vi "Main.vi"() -> ()   [LabVIEW 2020]
uses:
  System.Windows.Forms
  Global_Variable/Global.vi
  Global_Variable/A180648.vi
  <userlib>/_MGI/Menu Building/MenuTypes/MenuStrip/MGI_MenuStrip.lvclass
  <userlib>/_MGI/Menu Building/MenuItemStatusChange/MGI_MenuItemStatusChange.lvclass
  Libraries/S7/S7.lvlib
panel:
  out "状态":string
  out "客户软件版本号":string
  in  "Andon":enum32{"未选择", "缺料报警", "质量报警", "故障报警"}(radio)
  out "PLC":bool
  in  "菜单":refnum<k24>(container)
  in  "Result":string[][](table)
  out "逆向空载":bool
  out "试验计时":u16
  out "产品编号":string
  out "生产数量":i32
  out "合格数量":i32
  out "userStatus":string caption="用户状态"
  out "userName":string caption="用户名"
  out "connectionMode":string caption="联机类型"
  out "产品型号":string
  out "侧铆":bool
  out "轴承压装":bool
  out "振动NVH":bool
  out "磨合":bool
  out "备用试验2":bool
  out "传感器特性":bool
  out "电流特性":bool
  out "端铆":bool
  in  "更换产品":refnum<vi>
  out "提示信息":string
  out "错误":bool
  out "时间字符串":string
  out "日期字符串":string
  out "自动":bool=TRUE
  # "上柱管组件装配"
  # "试验项目"
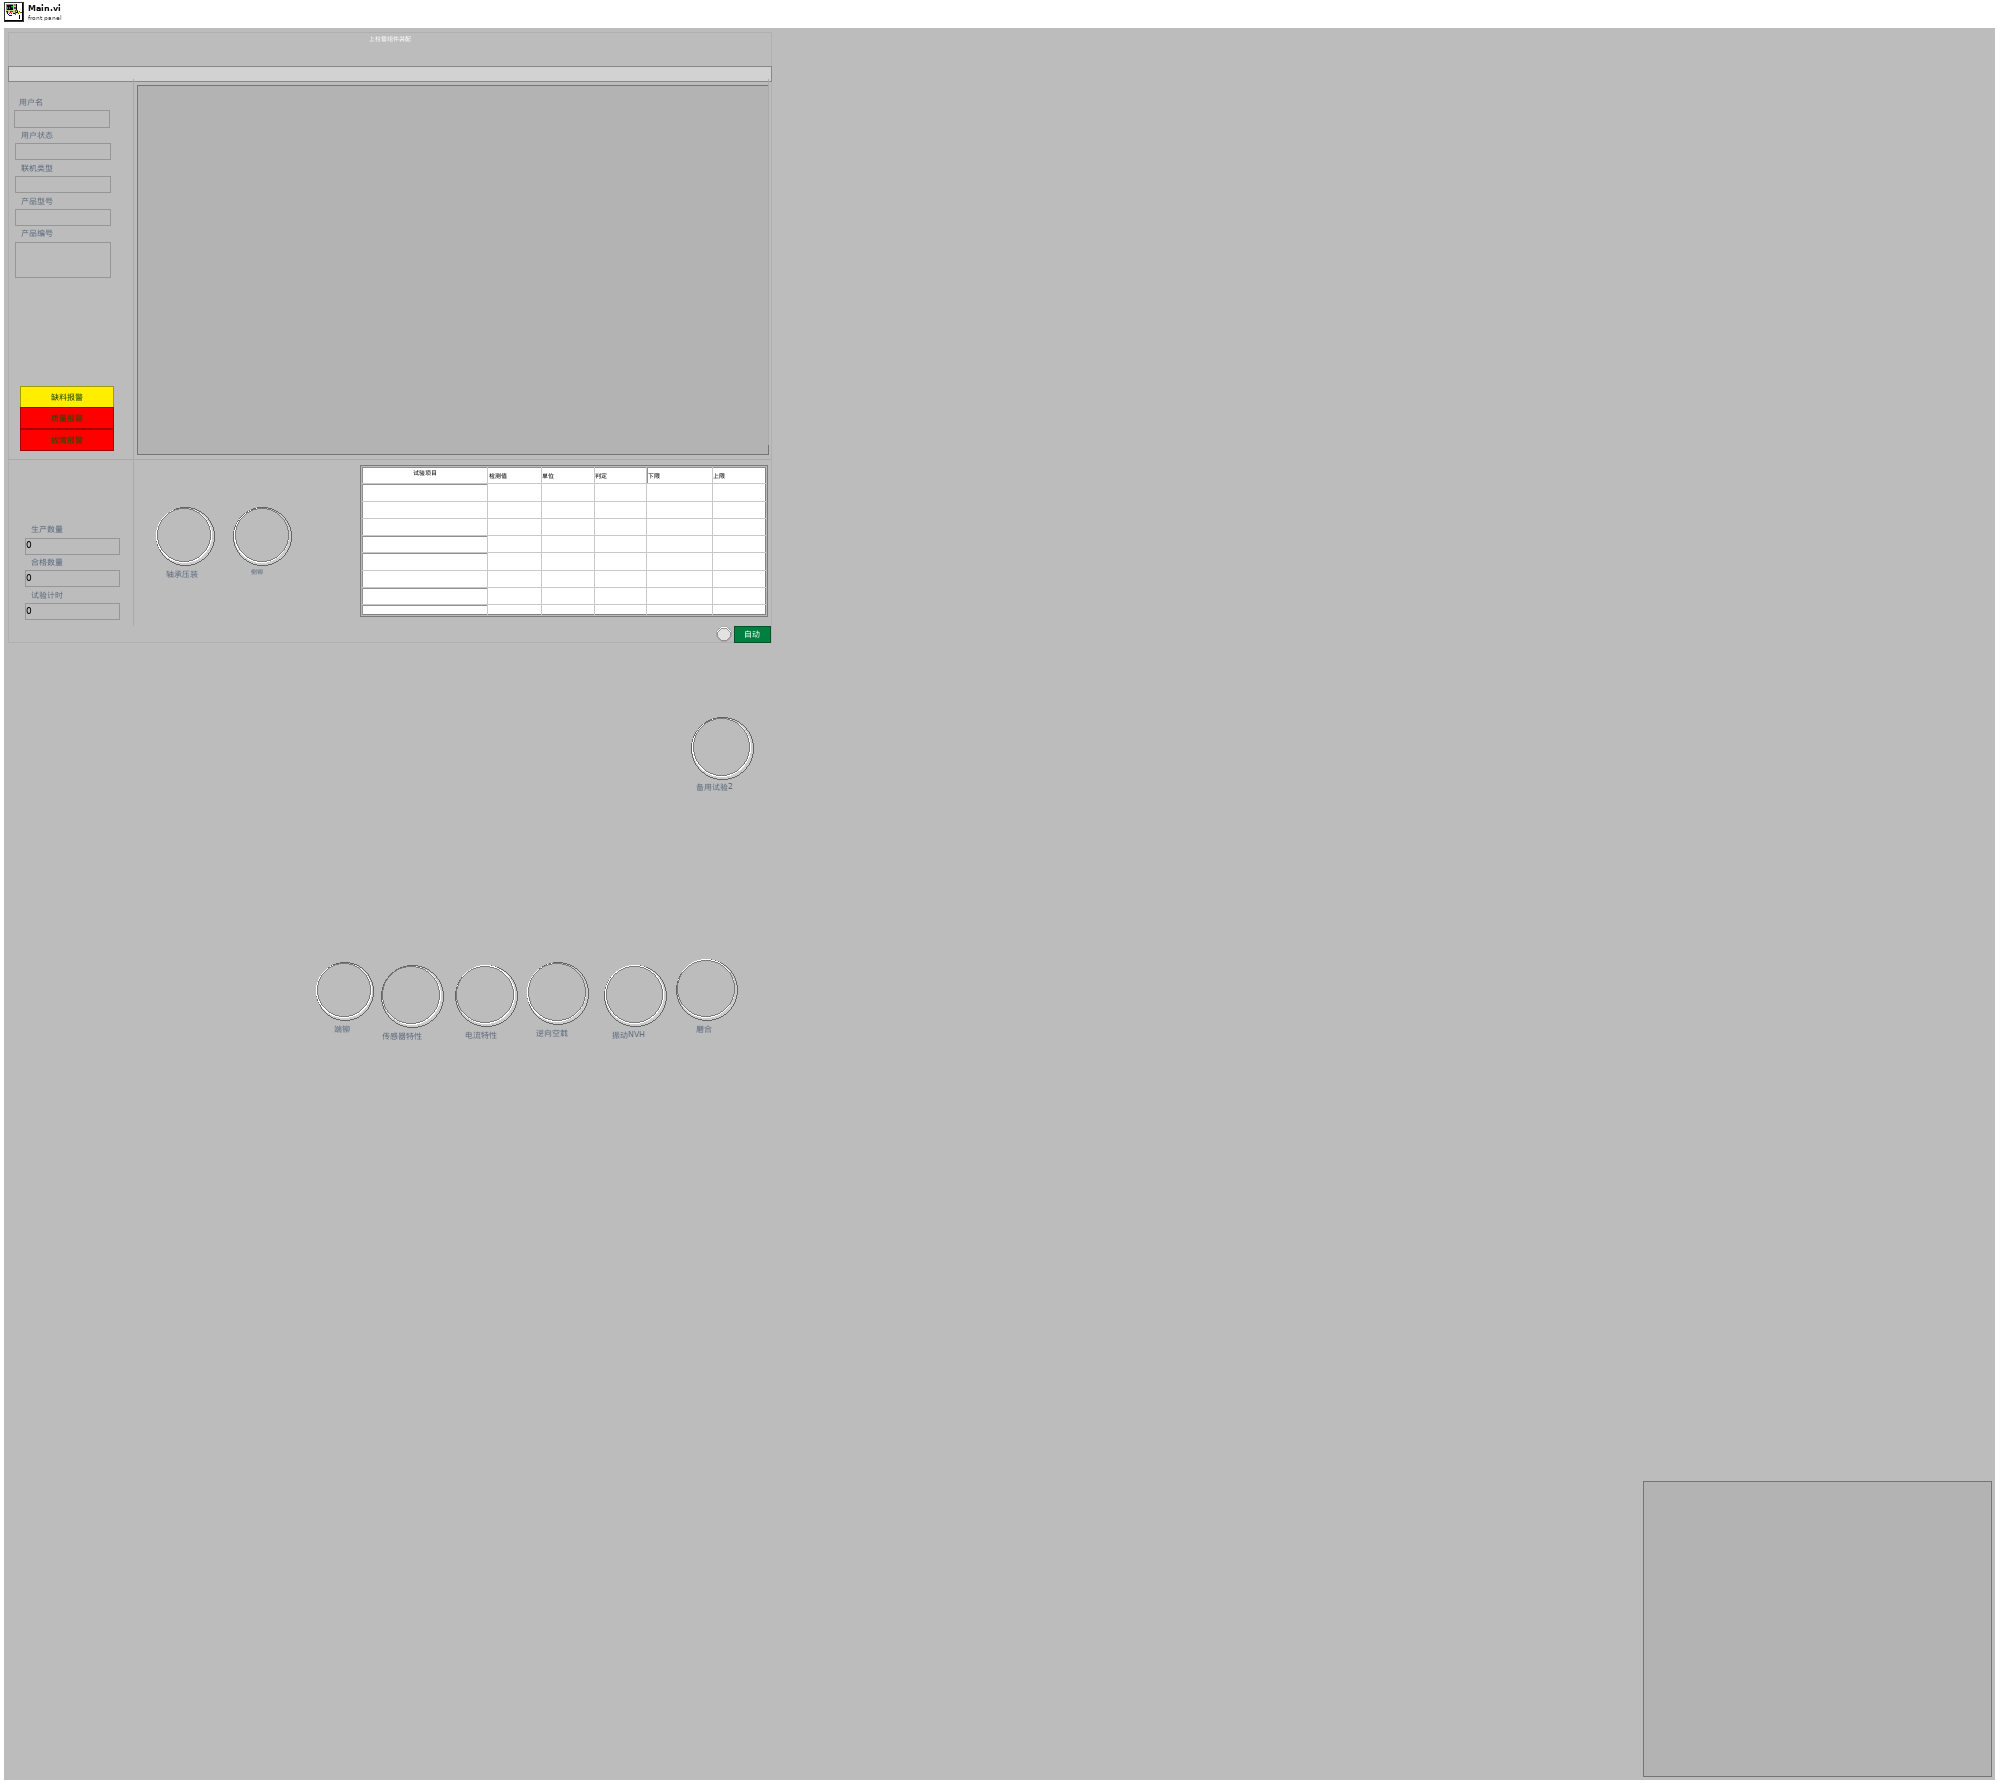
[diagram p1: front panel]
types:
  T1 = typedef "S7.lvlib/Broadcast Events--cluster.ctl" = cluster{"Module Did Init":refnum<user-event>, "Status Updated":refnum<user-event>, "Error Reported":refnum<user-event>, "Module Did Stop":refnum<user-event>, "Update Module Execution Status":refnum<user-event>}
  T2 = enum32{"轴承压装", "侧铆", "端铆", "力特性", "电流特性", "传感器特性", "逆向空载", "磨合"}
  T3 = enum32{"Invalid", "Standard", "Closed", "Hidden", "Minimized", "Maximized"}
  T4 = cluster{"设备名称":string, "操作人员":string, "设备状态":enum16{"设备离线", "设备正常", "设备缺料", "设备故障", "质量报警"}, "附加信息":string}
  T5 = enum32{"invalid app kind", "Development System", "Run Time System", "Student Edition", "Embedded LabVIEW", "Evaluation", "Custom"}
  T6 = cluster{"操作员编号":string, "操作员姓名":string, "操作员权限":string, "联机模式":enum16{"单机", "追溯"}}
  T7 = cluster{"Core":cluster{"Current VI Reference":refnum<vi>, "Close Panel on Exit?":bool}, "Your Boolean data":bool, "Your string data":string}
  T8 = cluster{"Current VI Reference":refnum<vi>, "Close Panel on Exit?":bool}
  T9 = cluster{"用户编号":string, "用户名":string, "用户密码(密文)":string, "用户权限":string}
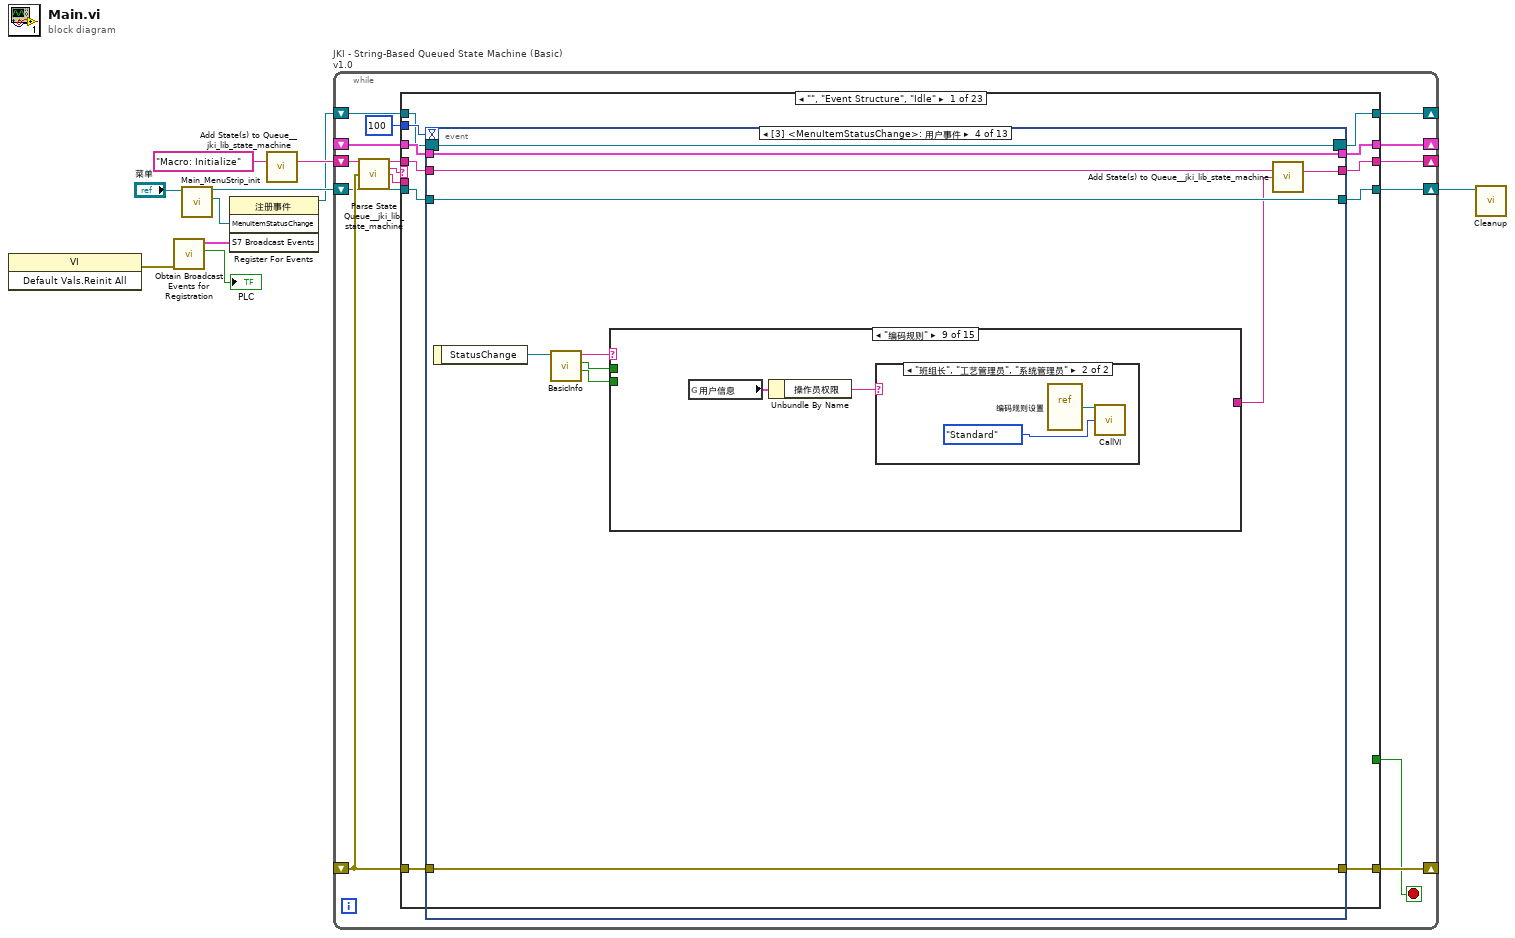
[diagram p0: block diagram]
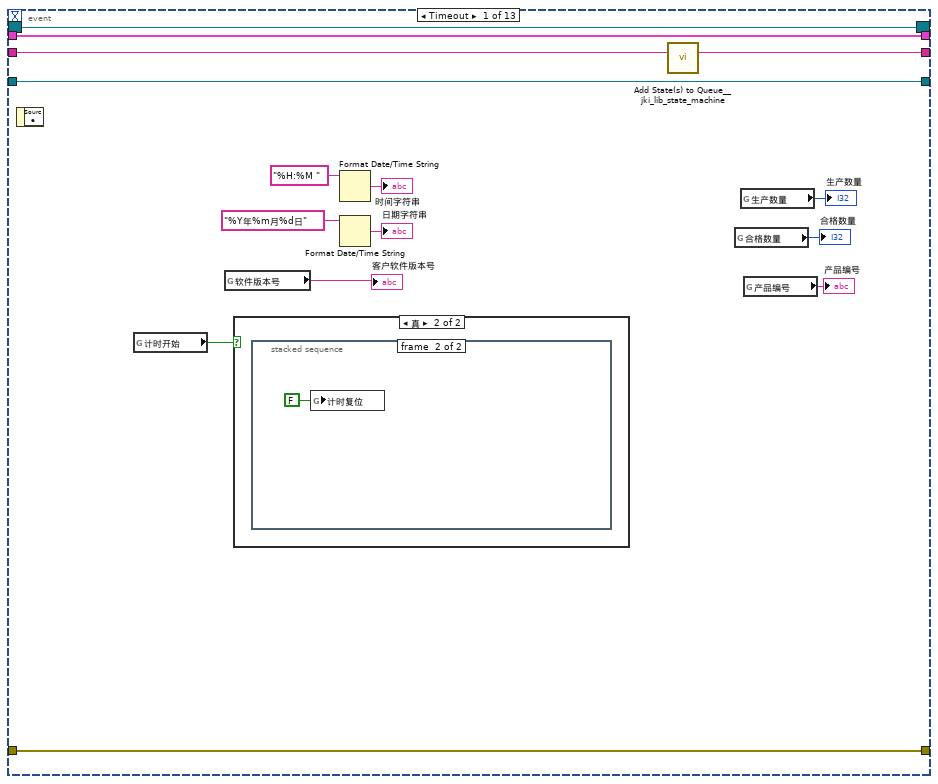
[diagram p2: hidden frame]
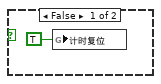
[diagram p3: hidden frame]
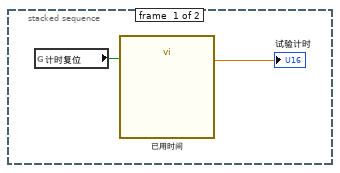
[diagram p4: hidden frame]
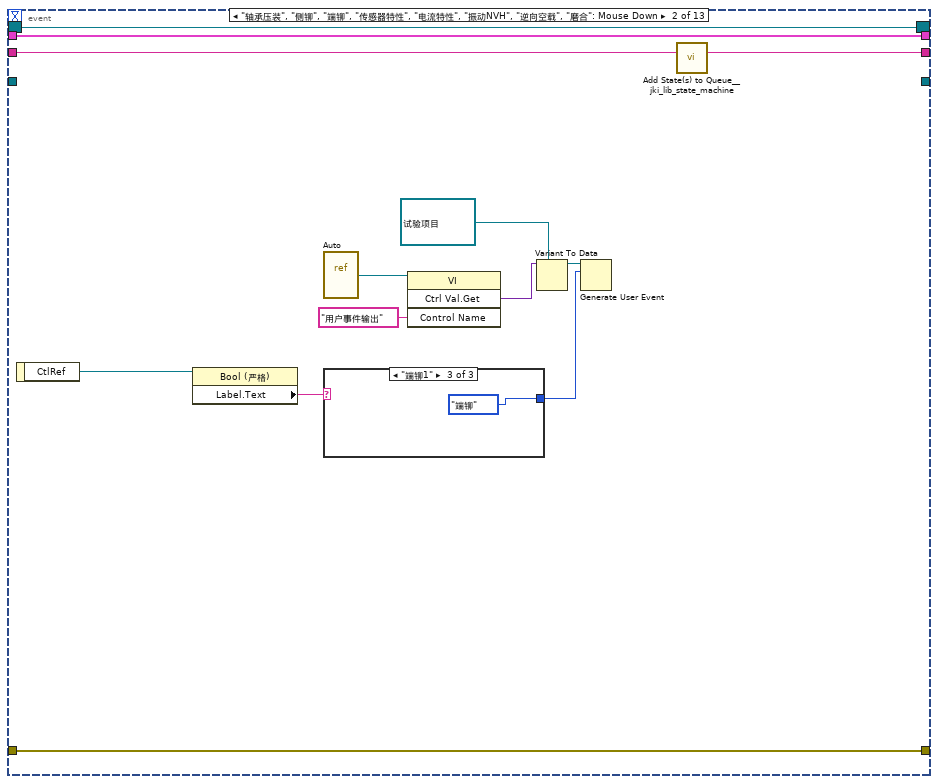
[diagram p5: hidden frame]
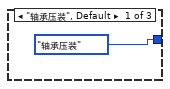
[diagram p6: hidden frame]
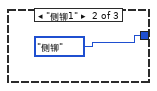
[diagram p7: hidden frame]
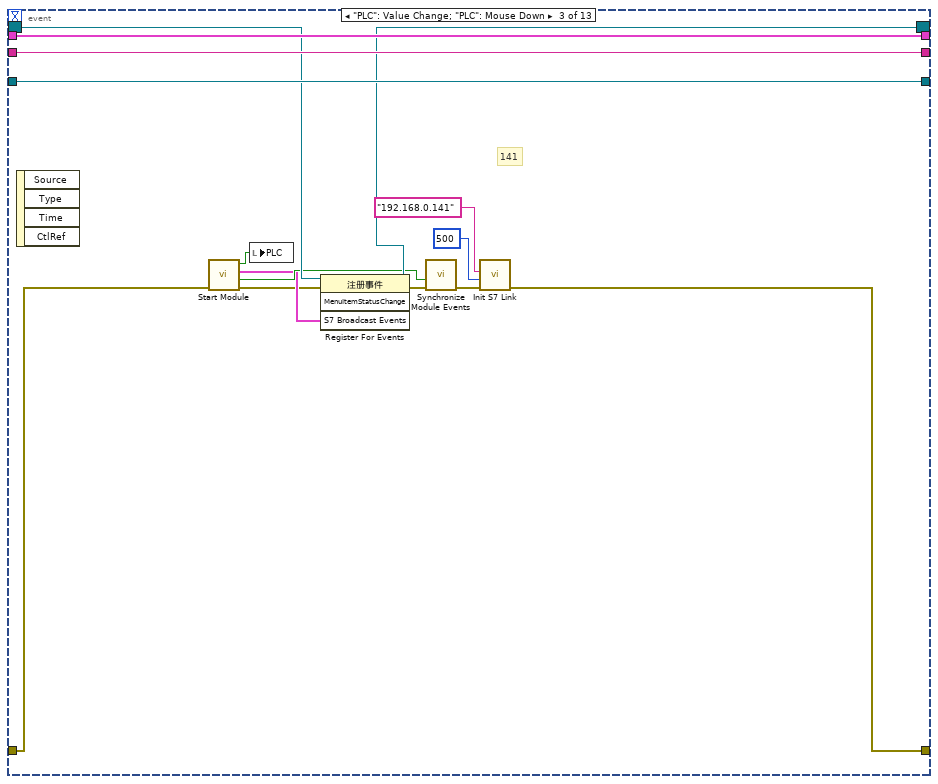
[diagram p8: hidden frame]
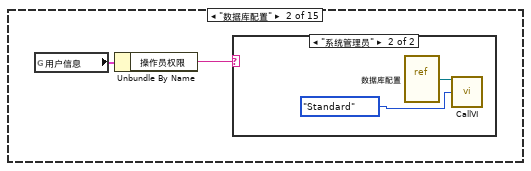
[diagram p10: hidden frame]
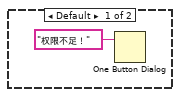
[diagram p11: hidden frame]
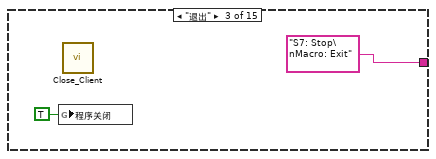
[diagram p12: hidden frame]
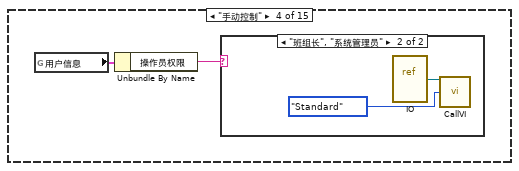
[diagram p13: hidden frame]
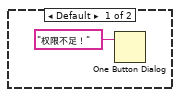
[diagram p14: hidden frame]
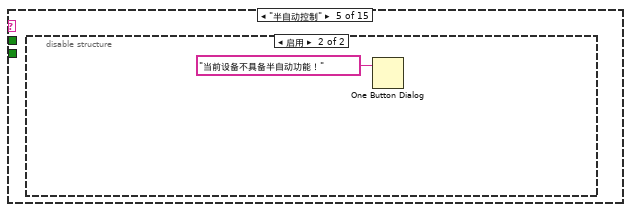
[diagram p15: hidden frame]
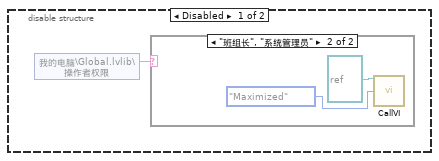
[diagram p16: hidden frame]
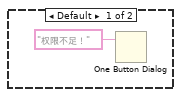
[diagram p17: hidden frame]
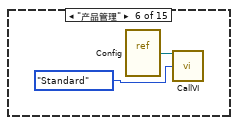
[diagram p18: hidden frame]
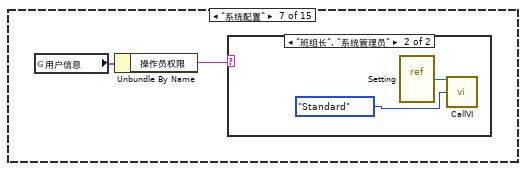
[diagram p19: hidden frame]
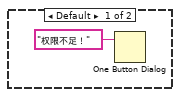
[diagram p20: hidden frame]
diagram:
  n1 = invoke class="VI" method="Default Vals.Reinit All"() -> (error out=w3:errorcluster)  [unwired: 3 in, 2 out]
  n2 = call "Obtain Broadcast Events for Registration.vi"("error in (no error)"=w3) -> ("Already running?"=→"PLC":bool, "S7 Broadcast Events"=w5:T1)  [unwired: 8 in, 1 out]
  n3 = call "Main_MenuStrip_init.vi"("MenuStrip"="菜单") -> ("MenuItemStatusChange"=w2:refnum<user-event>, "Menu out"=w7:refnum<class "MGI_MenuStrip.lvclass">)  [unwired: 9 in]
  n4 = register-events(w2, w5) -> (reference out=w1:refnum<event-registration>)  [unwired: 2 in, 1 out]
  n5 = call <vilib>:"Add State(s) to Queue__jki_lib_state_machine.vi"("State(s) in (\"\")"="Macro: Initialize") -> ("States Out"=w10:string)  [unwired: 14 in]
  n6 = while "JKI - String-Based Queued State Machine (Basic) v1.0" {
    shift-right: [w19] -> _
    shift-left: _ -> [w18]
    shift-right: [w21] -> _
    shift-left: _ -> [w16]
    shift-right: [w20] -> _
    shift-left: w10 -> [w22]
    shift-right: [w14] -> w6
    shift-left: w7 -> [w15]
    shift-right: [w12] -> _
    shift-left: w1 -> [w11]
    stop <- w13 stop-if-true
    n7 = call <vilib>:"Parse State Queue__jki_lib_state_machine.vi"("State Queue"=w22, "Error In (no error)"=w16) -> ("Remaining States"=w24:string, "Current State"=w25:string, "Arguments"=w23:string)  [unwired: 11 in]
    n8 = case shown="\"\", \"Event Structure\", \"Idle\"" w25 {
      selector: w25 -> [_ _ w273 _ _ _ _ _ _ _ _ _ _ _ _ _ _ _ _ _ _ _ _]
      tunnel: w24 -> [w36 w270 w277 w297 w305 w312 w318 w322 w328 w334 w340 w349 w360 w368 w374 w381 w395 w431 w439 w452 w480 w487 w499]
      tunnel: w23 -> [_ _ _ _ _ _ _ _ _ _ _ _ _ _ _ _ _ _ w434 w446 _ _ _]
      tunnel: w18 -> [w34 w267 w275 w288 w302 w310 w315 w323 w331 w337 w343 w346 _ w363 w371 w379 w393 w428 w437 w448 w477 w484 w496]
      tunnel: [w33 w268 w279 w294 errorcluster {"status"=FALSE, "code"=0, "source"=""} ("error out") w309 w316 w320 w326 w333 w339 w347 w357 w364 w372 w378 w391 w429 w435 w449 w478 w485 w497] -> w21
      tunnel: w16 -> [w32 w268 w278 w294 w301 w309 w316 w320 w327 w333 w339 w347 w357 w365 w372 w375 w391 w429 w436 w450 w478 w485 w497]
      tunnel: [w35 w269 w276 w296 w304 w311 w317 w322 w329 w335 w341 w348 w359 w367 w373 w380 w394 w430 w438 w451 w479 w486 w498] -> w20
      tunnel: [w31 w267 w275 w295 w302 w310 w315 w323 w331 w337 w343 w346 w358 w363 w371 w379 w393 w428 w437 w448 w477 w484 w496] -> w19
      tunnel: 100 ("Timeout") -> [w30 _ _ _ _ _ _ _ _ _ _ _ _ _ _ _ _ _ _ _ _ _ _]
      tunnel: w15 -> [w29 w266 w272 w285 w299 w308 w314 w321 w330 w336 w342 w345 w351 w362 w370 w377 w392 w427 w433 w445 w476 w482 w489]
      tunnel: [w28 w266 w272 w285 w299 w308 w314 w321 w330 w336 w342 w345 w351 w362 w370 w377 w392 w427 w433 w445 w476 w482 w489] -> w14
      tunnel: [_ _ _ _ _ TRUE _ _ _ _ _ _ _ _ _ _ _ _ _ _ _ _ _] -> w13
      tunnel: [w26 w265 w271 w284 w298 w306 w313 w324 w325 w332 w338 w344 w352 w361 w369 w376 w390 w424 w432 w444 w475 w481 w488] -> w12
      tunnel: w11 -> [w27 w265 w271 w284 w298 w306 w313 w324 w325 w332 w338 w344 w352 w361 w369 w376 w390 w424 w432 w444 w475 w481 w488]
      frame "", "Event Structure", "Idle" {
        n9 = event shown="[3] <MenuItemStatusChange>: 用户事件" {
          selector: w27 -> [w39 w64 w81 w87 w153 w160 w167 w174 w188 w200 w207 w215 _]
          dyn-events: [w39 w64 w80 w87 w153 w160 w167 w174 w188 w200 w207 w215 _] -> w26
          timeout: w30 -> [_ _ _ _ _ _ _ _ _ _ _ _ _]
          tunnel: w36 -> [w51 w67 w85 w96 w154 w161 w170 w177 w185 w204 w214 w217 w259]
          tunnel: [w50 w66 w85 w94 w155 w162 w171 w178 w186 w205 w213 w218 w259] -> w35
          tunnel: w34 -> [w49 w68 w86 w95 w157 w165 w172 w179 w187 w206 w211 w220 w260]
          tunnel: [w40 w65 w82 w97 w158 w163 w168 w180 w183 w203 w212 w219 w257] -> w33
          tunnel: w32 -> [w40 w65 w83 w97 w158 w163 w168 w181 w183 w203 w212 w219 w257]
          tunnel: [w49 w68 w86 w95 w157 w165 w172 w179 w187 w206 w211 w220 w260] -> w31
          tunnel: w29 -> [w38 _ w84 w90 w156 w164 w169 w176 w184 _ _ _ w258]
          tunnel: [w38 _ w84 w90 w156 w164 w169 w176 w184 _ _ _ w258] -> w28
          event Timeout {
            n10 = event-data() -> ()  [unwired: 1 in, 1 out]
            n11 = global read "Global.vi" "计时开始"() -> (w42:bool)
            n12 = global read "Global.vi" "软件版本号"() -> (→"客户软件版本号":string)
            n13 = case shown="真" w42 {
              frame False {
                n14 = global write "Global.vi" "计时复位"(TRUE ("计时复位")) -> ()
              }
              frame True {
                n15 = stacked-sequence {
                  frame #0 {
                    n16 = global read "Global.vi" "计时复位"() -> (w53:bool)
                    n17 = call "已用时间"("Reset"=w53) -> ("Elapsed Time (s)"=→"试验计时":dbl)  [unwired: 11 in, 7 out]
                  }
                  frame #1 {
                    n18 = global write "Global.vi" "计时复位"(FALSE ("计时复位")) -> ()
                  }
                }
              }
            }
            n19 = Format Date/Time String(time format string (%c)="%H:%M ") -> (date/time string=→"时间字符串":string)  [unwired: 2 in]
            n20 = Format Date/Time String(time format string (%c)="%Y年%m月%d日") -> (date/time string=→"日期字符串":string)  [unwired: 2 in]
            n21 = call <vilib>:"Add State(s) to Queue__jki_lib_state_machine.vi"("State(s) in (\"\")"=w51) -> ("States Out"=w50:string)  [unwired: 14 in]
            n22 = global read "Global.vi" "合格数量"() -> (→"合格数量":i32)
            n23 = global read "Global.vi" "生产数量"() -> (→"生产数量":i32)
            n24 = global read "Global.vi" "产品编号"() -> (→"产品编号":string)
          }
          event "轴承压装", "侧铆", "端铆", "传感器特性", "电流特性", "振动NVH", "逆向空载", "磨合": Mouse Down {
            w57 = refnum<user-event> refnum items=["轴承压装", "侧铆", "端铆", "力特性", "电流特性", "传感器特性", "逆向空载", "磨合"] ("用户事件输出")
            n25 = event-data() -> ("CtlRef"=w61:refnum<vi>)  [unwired: 1 in]
            n26 = property class="Bool (严格)"(reference=w61) -> ("Label.Text"=w60:string)  [unwired: 1 in, 2 out]
            n27 = vi-ref "Auto.vi"() -> (w63:refnum<vi>)
            n28 = case shown="\"端铆1\"" w60 {
              tunnel: [T2."轴承压装" ("试验项目") T2."侧铆" ("试验项目") T2."端铆" ("试验项目")] -> w59
              frame "轴承压装", Default {
              }
              frame "侧铆1" {
              }
              frame "端铆1" {
              }
            }
            n29 = invoke class="VI" method="Ctrl Val.Get"(reference=w63, "Control Name"="用户事件输出" ("控件名")) -> ("Get Control Value Variant"=w62:variant)  [unwired: 2 in, 3 out]
            n30 = Variant To Data(type=w57, Variant=w62) -> (data=w56:refnum<user-event>)  [unwired: 1 in, 1 out]
            n31 = Generate User Event(user event=w56, event data cluster=w59) -> ()  [unwired: 2 in, 2 out]
            n32 = call <vilib>:"Add State(s) to Queue__jki_lib_state_machine.vi"("State(s) in (\"\")"=w67) -> ("States Out"=w66:string)  [unwired: 14 in]
          }
          event "PLC": Value Change; "PLC": Mouse Down {
            # "141"
            n33 = event-data() -> ()  [unwired: 1 in, 4 out]
            n34 = call "Start Module.vi"("error in (no error)"=w83) -> ("error out"=w74:errorcluster, "Wait for Event Sync?"=w79:bool, "S7 Broadcast Events"=w78:T1, "Module Was Already Running?"=w77:bool)  [unwired: 7 in]
            n35 = local write "PLC"(w77) -> ()
            n36 = register-events(reference=w81, error in=w74, w78) -> (reference out=w80:refnum<event-registration>, error out=w73:errorcluster)  [unwired: 1 in]
            n37 = call "Synchronize Module Events.vi"("error in (no error)"=w73, "Wait for Event Sync?"=w79) -> ("error out"=w72:errorcluster)  [unwired: 9 in]
            n38 = call "Init S7 Link.vi"("error in (no error)"=w72, "超时"=500, "IP"="192.168.0.141") -> ("error out"=w82:errorcluster)  [unwired: 8 in]
          }
          event User Event {
            n39 = event-data() -> ("StatusChange"=w88:refnum<class "MGI_MenuItemStatusChange.lvclass">)  [unwired: 1 in]
            n40 = call <userlib>:"BasicInfo.vi"("MGI_MenuItemStatusChange in"=w88) -> ("Enabled?"=w91:bool, "Checked?"=w92:bool, "Tag"=w93:string)  [unwired: 7 in, 1 out]
            n41 = case shown="\"编码规则\"" w93 {
              tunnel: w92 -> [_ _ _ _ _ _ _ _ _ _ _ _ _ _ _]
              tunnel: w91 -> [_ _ _ _ _ _ _ _ _ _ _ _ _ _ _]
              tunnel: [_ _ "S7: Stop\nMacro: Exit" _ _ _ _ _ _ _ _ _ _ _ _] -> w89
              frame "假", Default {
              }
              frame "数据库配置" {
                n42 = global read "用户信息.vi" "用户信息"() -> (w99:T6)
                n43 = Unbundle By Name(w99) -> ("操作员权限"=w98:string)
                n44 = case shown="\"系统管理员\"" w98 {
                  frame Default {
                    n45 = One Button Dialog(message="权限不足！" ("消息")) -> ()  [unwired: 1 in, 1 out]
                  }
                  frame "系统管理员" {
                    n46 = vi-ref "数据库配置.vi"() -> (w102:refnum<vi>)
                    n47 = call "CallVI.vi"("VI引用"=w102, "状态"=T3."Standard") -> ()  [unwired: 12 in, 2 out]
                  }
                }
              }
              frame "退出" {
                n48 = global write "Global.vi" "程序关闭"(TRUE ("程序关闭")) -> ()
                n49 = call "Close_Client.vi"() -> ()  [unwired: 12 in]
              }
              frame "手动控制" {
                n50 = global read "用户信息.vi" "用户信息"() -> (w106:T6)
                n51 = Unbundle By Name(w106) -> ("操作员权限"=w105:string)
                n52 = case shown="\"班组长\", \"系统管理员\"" w105 {
                  frame Default {
                    n53 = One Button Dialog(message="权限不足！" ("消息")) -> ()  [unwired: 1 in, 1 out]
                  }
                  frame "班组长", "系统管理员" {
                    n54 = vi-ref "IO.vi"() -> (w109:refnum<vi>)
                    n55 = call "CallVI.vi"("VI引用"=w109, "状态"=T3."Standard") -> ()  [unwired: 12 in, 2 out]
                  }
                }
              }
              frame "半自动控制" {
                n56 = disable-structure shown="启用" {
                  frame Disabled {
                    n57 = shared-variable "我的电脑\\Global.lvlib\\操作者权限"() -> (w110:string)  [unwired: 1 in, 1 out]
                    n58 = case shown="\"班组长\", \"系统管理员\"" w110 {
                      frame Default {
                        n59 = One Button Dialog(message="权限不足！" ("消息")) -> ()  [unwired: 1 in, 1 out]
                      }
                      frame "班组长", "系统管理员" {
                        n60 = call "CallVI.vi"("VI引用"=refnum<vi> refnum, "状态"=T3."Maximized") -> ()  [unwired: 12 in, 2 out]
                      }
                    }
                  }
                  frame Enabled {
                    n61 = One Button Dialog(message="当前设备不具备半自动功能！" ("消息")) -> ()  [unwired: 1 in, 1 out]
                  }
                }
              }
              frame "产品管理" {
                n62 = vi-ref "Config.vi"() -> (w116:refnum<vi>)
                n63 = call "CallVI.vi"("VI引用"=w116, "状态"=T3."Standard") -> ()  [unwired: 12 in, 2 out]
              }
              frame "系统配置" {
                n64 = global read "用户信息.vi" "用户信息"() -> (w118:T6)
                n65 = Unbundle By Name(w118) -> ("操作员权限"=w117:string)
                n66 = case shown="\"班组长\", \"系统管理员\"" w117 {
                  frame Default {
                    n67 = One Button Dialog(message="权限不足！" ("消息")) -> ()  [unwired: 1 in, 1 out]
                  }
                  frame "班组长", "系统管理员" {
                    n68 = vi-ref "Setting.vi"() -> (w121:refnum<vi>)
                    n69 = call "CallVI.vi"("VI引用"=w121, "状态"=T3."Standard") -> ()  [unwired: 12 in, 2 out]
                  }
                }
              }
              frame "用户管理" {
                n70 = global read "用户信息.vi" "用户信息"() -> (w123:T6)
                n71 = Unbundle By Name(w123) -> ("操作员权限"=w122:string)
                n72 = case shown="\"系统管理员\"" w122 {
                  frame Default {
                    n73 = One Button Dialog(message="权限不足！" ("消息")) -> ()  [unwired: 1 in, 1 out]
                  }
                  frame "系统管理员" {
                    n74 = vi-ref "User_manager.vi"() -> (w126:refnum<vi>)
                    n75 = call "CallVI.vi"("VI引用"=w126, "状态"=T3."Standard") -> ()  [unwired: 12 in, 2 out]
                  }
                }
              }
              frame "编码规则" {
                n76 = global read "用户信息.vi" "用户信息"() -> (w128:T6)
                n77 = Unbundle By Name(w128) -> ("操作员权限"=w127:string)
                n78 = case shown="\"班组长\", \"工艺管理员\", \"系统管理员\"" w127 {
                  frame Default {
                    n79 = One Button Dialog(message="权限不足！" ("消息")) -> ()  [unwired: 1 in, 1 out]
                  }
                  frame "班组长", "工艺管理员", "系统管理员" {
                    n80 = vi-ref "编码规则设置.vi"() -> (w131:refnum<vi>)
                    n81 = call "CallVI.vi"("VI引用"=w131, "状态"=T3."Standard") -> ()  [unwired: 12 in, 2 out]
                  }
                }
              }
              frame "易损件管理" {
                n82 = vi-ref "易损件管理.vi"() -> (w133:refnum<vi>)
                n83 = call "CallVI.vi"("VI引用"=w133, "状态"=T3."Standard") -> ()  [unwired: 12 in, 2 out]
              }
              frame "物料批次管理" {
                n84 = vi-ref "批次管理.vi"() -> (w135:refnum<vi>)
                n85 = call "CallVI.vi"("VI引用"=w135, "状态"=T3."Standard") -> ()  [unwired: 12 in, 2 out]
              }
              frame "报表" {
                n86 = call "文件对话框"("start path"=path "D:/report", "prompt"="打开报表", "pattern (all files)"="*.doc;*.docx", "pattern label"="Word 文档") -> ("selected path"=w136:path, "error out"=w137:errorcluster)  [unwired: 8 in, 2 out]
                n87 = case shown="无错误" w137 {
                  selector: w137 -> [w143 w145]
                  tunnel: w136 -> [w144 _]
                  frame No Error {
                    w142 = 1 items=["Normal", "Maximize", "Minimize"] ("cpubbs_WindowState")
                    n88 = call "Open_Word.vi"("File Path"=w144, "cpubbs_WindowState"=w142, "错误输入（无错误）"=w143) -> ()  [unwired: 12 in, 1 out]
                  }
                  frame Error {
                    n89 = call <vilib>:"Clear Errors.vi"("error in (no error)"=w145) -> ()  [unwired: 5 in, 2 out]
                  }
                }
              }
              frame "报警信息" {
                n90 = vi-ref "报警信息.vi"() -> (w147:refnum<vi>)
                n91 = call "CallVI.vi"("VI引用"=w147, "状态"=T3."Standard") -> ()  [unwired: 12 in, 2 out]
              }
              frame "关于" {
                n92 = vi-ref "About.vi"() -> (w149:refnum<vi>)
                n93 = call "CallVI.vi"("VI引用"=w149, "状态"=T3."Standard") -> ()  [unwired: 12 in, 2 out]
              }
              frame "操作演示" {
                n94 = call <vilib>:"Application Directory.vi"() -> ("Application Directory"=w152:path)
                n95 = Build Path(base path=w152, name or relative path="操作演示" ("名称或相对路径")) -> (appended path=w151:path)
                n96 = call "自动播放ppt.vi"("路径"=w151) -> ()  [unwired: 10 in, 1 out]
              }
            }
            n97 = call <vilib>:"Add State(s) to Queue__jki_lib_state_machine.vi"("State(s) in (\"\")"=w96, "State(s) at Back (\"\")"=w89) -> ("States Out"=w94:string)  [unwired: 13 in]
          }
          event User Event {
            n98 = event-data() -> ("Init?"=w159:bool)  [unwired: 1 in, 1 out]
            n99 = local write "PLC"(w159) -> ()
            n100 = call <vilib>:"Add State(s) to Queue__jki_lib_state_machine.vi"("State(s) in (\"\")"=w154) -> ("States Out"=w155:string)  [unwired: 14 in]
          }
          event User Event {
            n101 = event-data() -> ("Running?"=w166:bool)  [unwired: 1 in]
            n102 = local write "PLC"(w166) -> ()
            n103 = call <vilib>:"Add State(s) to Queue__jki_lib_state_machine.vi"("State(s) in (\"\")"=w161) -> ("States Out"=w162:string)  [unwired: 14 in]
          }
          event User Event {
            n104 = event-data() -> ()  [unwired: 1 in, 7 out]
            n105 = local write "PLC"(FALSE ("PLC")) -> ()
            n106 = call <vilib>:"Add State(s) to Queue__jki_lib_state_machine.vi"("State(s) in (\"\")"=w170) -> ("States Out"=w171:string)  [unwired: 14 in]
          }
          event User Event {
            n107 = event-data() -> ("Error"=w182:errorcluster)  [unwired: 1 in]
            n108 = Merge Errors(w182, w181) -> (w180:errorcluster)
            n109 = call <vilib>:"Add State(s) to Queue__jki_lib_state_machine.vi"("State(s) in Front (\"\")"="S7: Initialize\nIdle", "State(s) in (\"\")"=w177) -> ("States Out"=w178:string)  [unwired: 13 in]
          }
          event "自动": Mouse Down {
            n110 = event-data() -> ()  [unwired: 1 in, 1 out]
            n111 = disable-structure shown="禁用" {
              frame Disabled {
                n112 = local read "自动"() -> (w189:bool)
                n113 = case shown="真" w189 {
                  frame False {
                    n114 = call "设备状态.vi"() -> ("Status_Read"=w190:i16)  [unwired: 11 in]
                    n115 = case shown="5" w190 {
                      frame 0, Default {
                        n116 = One Button Dialog(message="请复位！" ("消息")) -> ()  [unwired: 1 in, 1 out]
                      }
                      frame 5 {
                        n117 = vi-ref "Auto.vi"() -> (w194:refnum<vi>)
                        n118 = invoke class="VI" method="Ctrl Val.Set"(reference=w194, "Control Name"="STEP" ("控件名"), "Value"="进入自动" ("控件名")) -> ()  [unwired: 2 in, 5 out]
                      }
                    }
                  }
                  frame True {
                    n119 = Two Button Dialog(message="确定要退出自动？" ("消息")) -> (T button?=w195:bool)  [unwired: 2 in]
                    n120 = case shown="真" w195 {
                      frame False {
                      }
                      frame True {
                        n121 = vi-ref "Auto.vi"() -> (w199:refnum<vi>)
                        n122 = invoke class="VI" method="Ctrl Val.Set"(reference=w199, "Control Name"="STEP" ("控件名"), "Value"="退出自动" ("控件名")) -> ()  [unwired: 2 in, 5 out]
                      }
                    }
                  }
                }
              }
              frame Enabled {
              }
            }
            n123 = call <vilib>:"Add State(s) to Queue__jki_lib_state_machine.vi"("State(s) in (\"\")"=w185) -> ("States Out"=w186:string)  [unwired: 14 in]
          }
          event "错误": Mouse Down {
            n124 = event-data() -> ()  [unwired: 1 in, 8 out]
            n125 = vi-ref "报警信息.vi"() -> (w202:refnum<vi>)
            n126 = call "CallVI.vi"("VI引用"=w202, "状态"=T3."Standard") -> ()  [unwired: 12 in, 2 out]
            n127 = call <vilib>:"Add State(s) to Queue__jki_lib_state_machine.vi"("State(s) in (\"\")"=w204) -> ("States Out"=w205:string)  [unwired: 14 in]
          }
          event Panel Close? {
            n128 = event-data() -> ()  [unwired: 1 in, 1 out]
            n129 = global write "Global.vi" "程序关闭"(TRUE ("程序关闭")) -> ()
            n130 = call <vilib>:"Add State(s) to Queue__jki_lib_state_machine.vi"("State(s) in Front (\"\")"="S7: Stop\nMacro: Exit", "State(s) in (\"\")"=w214) -> ("States Out"=w213:string)  [unwired: 13 in]
            n131 = event-data("Discard?"=TRUE) -> ()  [unwired: 1 in, 1 out]
          }
          event "更换产品": Value Change {
            n132 = event-data() -> ("NewVal"=w216:refnum<vi>)  [unwired: 1 in, 5 out]
            n133 = stacked-sequence {
              tunnel: w216 -> [w221]
              frame #0 {
                n134 = stacked-sequence {
                  tunnel: w221 -> [w229 _]
                  frame #0 {
                    n135 = disable-structure shown="禁用" {
                      disable-tunnel: w229 -> [w231 _]
                      frame Disabled {
                        n136 = control-ref of="子面板"() -> (w230:refnum<vi>)
                        n137 = call "Call_SubPanal.vi"("VI引用句柄"=w231, "SubPnl引用句柄"=w230) -> ()  [unwired: 9 in, 1 out]
                      }
                      frame Enabled {
                      }
                    }
                    n138 = vi-ref "Auto.vi"() -> (w228:refnum<vi>)
                    n139 = invoke class="VI" method="Ctrl Val.Get"(reference=w228, "Control Name"="产品变更_Event" ("控件名")) -> ("Get Control Value Variant"=w226:variant)  [unwired: 2 in, 3 out]
                    n140 = global read "Global.vi" "产品型号"() -> (w223:string)
                    n141 = Variant To Data(type=refnum<user-event> refnum ("产品变更_Event"), Variant=w226) -> (data=w224:refnum<user-event>, error out=w222:errorcluster)  [unwired: 1 in]
                    n142 = Generate User Event(user event=w224, event data cluster=w223, error in=w222) -> ()  [unwired: 1 in, 2 out]
                    n143 = local write "产品型号"(w223) -> ()
                  }
                  frame #1 {
                    n144 = control-ref of="轴承压装"() -> (w232:refnum<vi>)
                    n145 = control-ref of="侧铆"() -> (w233:refnum<vi>)
                    n146 = control-ref of="端铆"() -> (w234:refnum<vi>)
                    n147 = global read "Global.vi" "试验项目"() -> (w237:bool[])
                    n148 = Build Array(w232, w233, w234) -> (w236:refnum<vi>[])
                    n149 = for {
                      tunnel: w236 -> [w241] mode=indexing
                      tunnel: w237 -> [w242] mode=indexing
                      shift-right: [w238] -> _
                      shift-left: 2000 -> [w239]
                      i -> [w240]
                      n150 = case shown="真" w242 {
                        tunnel: w241 -> [w243 w251]
                        tunnel: w240 -> [_ _]
                        tunnel: w239 -> [w245 w248]
                        tunnel: [w245 w246] -> w238
                        frame False {
                          n151 = property class="Bool (严格)"(reference=w243, "Top"=2000) -> ()  [unwired: 1 in, 2 out]
                        }
                        frame True {
                          n152 = Add(x=w248, y=120) -> (x+y=w246:i32)
                          n153 = Bundle(w246, 1235) -> (w249:cluster{i32, i32})  [unwired: 1 in]
                          n154 = property class="Bool (严格)"(reference=w251, "Position"=w249) -> ()  [unwired: 1 in, 2 out]
                        }
                      }
                    }
                  }
                }
              }
            }
            n155 = call <vilib>:"Add State(s) to Queue__jki_lib_state_machine.vi"("State(s) in (\"\")"=w217) -> ("States Out"=w218:string)  [unwired: 14 in]
          }
          event "Andon": Value Change {
            n156 = event-data() -> ("NewVal"=w256:enum32{"未选择", "缺料报警", "质量报警", "故障报警"})  [unwired: 1 in]
            n157 = case shown="\"未选择\", 默认" w256 {
              tunnel: [enum16{"设备离线", "设备正常", "设备缺料", "设备故障", "质量报警"}."设备正常" ("设备状态") enum16{"设备离线", "设备正常", "设备缺料", "设备故障", "质量报警"}."设备缺料" ("设备状态") enum16{"设备离线", "设备正常", "设备缺料", "设备故障", "质量报警"}."质量报警" ("设备状态") enum16{"设备离线", "设备正常", "设备缺料", "设备故障", "质量报警"}."设备故障" ("设备状态")] -> w254
              frame "未选择", Default {
              }
              frame "缺料报警" {
              }
              frame "质量报警" {
              }
              frame "故障报警" {
              }
            }
            n158 = local read "userName"() -> (w253:string)
            n159 = Bundle By Name(cluster=T4 {"设备名称"="最终性能试验台1", "操作人员"="", "设备状态"=enum."设备离线", "附加信息"=""} ("设备信息"), "操作人员"=w253, "设备状态"=w254) -> (w252:T4)
            n160 = call "Change_Client.vi"("设备信息"=w252) -> ()  [unwired: 10 in, 1 out]
          }
        }
      }
      frame "---------- Core ----------" {
        n161 = call <vilib>:"Add State(s) to Queue__jki_lib_state_machine.vi"("State(s) in (\"\")"=w270) -> ("States Out"=w269:string)  [unwired: 14 in]
      }
      frame Default {
        w282 = 42 items=["No error", "Argument error", "Memory is full", "Out of zone", "End of file", "File already open", "Generic file I/O error", "File not found", "File permission error", "Disk is full", "Duplicate path", "Too many files open", "System feature not enabled", "Resource file not found", "Cannot add resource", "Resource not found", "Image not found", "Image memory error", "Pen does not exist", "Config type invalid", "Config token not found", "Config parse error", "Config memory error", "Bad external code format", "Bad external code offset", "External code not present", "Null window", "Destroy window error", "Null menu", "Print aborted", "Bad print record", "Print driver error", "Windows error during printing", "Memory error during printing", "Print dialog error", "Generic print error", "Invalid device refnum", "Device not found", "Device parameter error", "Device unit error", "Cannot open device", "Device call aborted", "Generic error", "Cancelled by user", "Object ID too low", "Object ID too high", "Object not in heap", "Unknown heap", "Unknown object (invalid DefProc)", "Unknown object (DefProc not in table)", "Message out of range", "Invalid (null) method", "Unknown message", "Manager call not supported", "Bad address", "Network operation in progress", "Network operation timed out", "Connection is busy", "Network attribute not supported", "Network error", "Address in use", "System out of memory", "Connection aborted", "Connection refused", "Not connected", "Already connected", "Connection closed", "Initialization error (interapplication manager)", "Bad occurrence", "Wait on unbound occurrence handler", "Occurrence queue overflow", "Datalog type conflict", "Unused", "Unrecognized type (interapplication manager)", "Memory corrupt", "Failed to make temporary DLL", "Old CIN version", "Drag socket not found", "Failed to load drop-object", "Failed to register OLE object", "Failed to release OLE object", "Format specifier type mismatch", "Unknown format specifier", "Too few format specifiers", "Too many format specifiers", "Scan failed", "Newer CIN version", "Error converting to variant", "Runtime menu error", "Password tampered", "Variant attribute not found", "Incompatible variant data type", "Event data is not available", "Event Store is not present", "Occurrence is not found", "Event Queue is not created", "Event info is not available", "Refnum passed is NULL", "Error retrieving Class GUID", "Error retrieving CoClass GUID", "Error retrieving TypeLib GUID.", "Bad built application magic bytes.", "Specific driver is different from the specific driver associated with the Logical Name.", "There is no session opened to the class driver.", "Max Error", "MAX - Error with config objects", "MAX - Error loading configuration", "MAX - Group not supported"]
        # "Current State"
        n162 = Format Into String(format string="Software Exception: Unhandled State \"%s\"." ("message"), error in=w278, w273) -> (resulting string=w281:string, error out=w280:errorcluster)  [unwired: 1 in]
        n163 = call <vilib>:"Error Cluster From Error Code.vi"("show call chain? (False)"=TRUE, "error in (no error)"=w280, "error message (\"\")"=w281, "error code (0)"=w282) -> ("error out"=w279:errorcluster)  [unwired: 5 in]
        n164 = call <vilib>:"Add State(s) to Queue__jki_lib_state_machine.vi"("State(s) in (\"\")"=w277) -> ("States Out"=w276:string)  [unwired: 14 in]
      }
      frame "Initialize Core Data" {
        # "originally closed?"
        # "exe?"
        n165 = property class="VI"() -> ("Front Panel.Open"=w293:bool)  [unwired: 2 in, 2 out]
        n166 = property class="App"() -> ("App.Kind"=w292:T5)  [unwired: 2 in, 2 out]
        n167 = control-ref of="Current VI Reference"() -> (w286:refnum<vi>)
        n168 = Not(x=w293) -> (.not. x?=w290:bool)
        n169 = Equal?(x=w292, y=T5."Run Time System" ("Application:Kind")) -> (x = y?=w289:bool)
        n170 = Or(x=w290, y=w289) -> (x .or. y?=w287:bool)
        n171 = Bundle By Name(cluster=w288, "Core.Current VI Reference"=w286, "Core.Close Panel on Exit?"=w287) -> (w295:T7)
        n172 = call <vilib>:"Add State(s) to Queue__jki_lib_state_machine.vi"("State(s) in (\"\")"=w297) -> ("States Out"=w296:string)  [unwired: 14 in]
      }
      frame "Error Handler" {
        n173 = call <vilib>:"General Error Handler.vi"("error in (no error)"=w301) -> ()  [unwired: 10 in, 5 out]
        n174 = call <vilib>:"Add State(s) to Queue__jki_lib_state_machine.vi"("State(s) in Front (\"\")"="/* Post Error States", "State(s) in (\"\")"=w305) -> ("States Out"=w304:string)  [unwired: 13 in]
      }
      frame "Exit" {
        n175 = call <vilib>:"Add State(s) to Queue__jki_lib_state_machine.vi"("State(s) in (\"\")"=w312) -> ("States Out"=w311:string)  [unwired: 14 in]
        n176 = Quit LabVIEW() -> ()  [unwired: 1 in]
      }
      frame "--------- Library --------" {
        n177 = call <vilib>:"Add State(s) to Queue__jki_lib_state_machine.vi"("State(s) in (\"\")"=w318) -> ("States Out"=w317:string)  [unwired: 14 in]
      }
      frame "S7: Initialize" {
        n178 = property on="PLC" class="Bool (严格)"("Val(Sgnl)"=FALSE ("值(信号)")) -> ()  [unwired: 2 in, 2 out]
      }
      frame "S7: Stop" {
        n179 = call "Stop Module.vi"("error in (no error)"=w327) -> ("error out"=w326:errorcluster)  [unwired: 10 in]
        n180 = call <vilib>:"Add State(s) to Queue__jki_lib_state_machine.vi"("State(s) in (\"\")"=w328) -> ("States Out"=w329:string)  [unwired: 14 in]
      }
      frame "CAN: Start" {
        n181 = call <vilib>:"Add State(s) to Queue__jki_lib_state_machine.vi"("State(s) in (\"\")"=w334) -> ("States Out"=w335:string)  [unwired: 14 in]
      }
      frame "CAN: Stop" {
        n182 = call <vilib>:"Add State(s) to Queue__jki_lib_state_machine.vi"("State(s) in (\"\")"=w340) -> ("States Out"=w341:string)  [unwired: 14 in]
      }
      frame "---------- Data ----------" {
        n183 = call <vilib>:"Add State(s) to Queue__jki_lib_state_machine.vi"("State(s) in (\"\")"=w349) -> ("States Out"=w348:string)  [unwired: 14 in]
      }
      frame "Data: Initialize" {
        w354 = T8 {"Current VI Reference"=refnum, "Close Panel on Exit?"=FALSE}  # Core
        w356 = TRUE  # Your Boolean data
        w355 = ""  # Your string data
        n184 = global write "Global.vi" "程序关闭"(FALSE ("程序关闭")) -> ()
        n185 = global write "Global.vi" "计时开始"(FALSE ("计时结束")) -> ()
        n186 = Bundle("Core"=w354, "Your Boolean data"=w356, "Your string data"=w355) -> (w358:T7)  [unwired: 1 in]
        n187 = call <vilib>:"Add State(s) to Queue__jki_lib_state_machine.vi"("State(s) in (\"\")"=w360) -> ("States Out"=w359:string)  [unwired: 14 in]
      }
      frame "Data: Cleanup" {
        n188 = Unbundle By Name(w363) -> ("Core.Current VI Reference"=w366:refnum<vi>)
        n189 = Close Reference(reference=w366, error in (no error)=w365) -> (error out=w364:errorcluster)
        n190 = call <vilib>:"Add State(s) to Queue__jki_lib_state_machine.vi"("State(s) in (\"\")"=w368) -> ("States Out"=w367:string)  [unwired: 14 in]
      }
      frame "---------- UI ----------" {
        # "Do not put any code in this frame.\n(It is a separator no-op. You can make a copy of this frame to create a new UI frame)"
        n191 = call <vilib>:"Add State(s) to Queue__jki_lib_state_machine.vi"("State(s) in (\"\")"=w374) -> ("States Out"=w373:string)  [unwired: 14 in]
      }
      frame "UI: Initialize" {
        n192 = disable-structure shown="启用" {
          disable-tunnel: [w384 _] -> w378
          disable-tunnel: w375 -> [w382 _]
          frame Enabled {
            n193 = vi-ref "Auto.vi"() -> (w383:refnum<vi>)
            n194 = invoke on="子面板" class="SubPnl" method="Insert VI"(error in=w382, "VI Ref"=w383) -> (error out=w387:errorcluster)  [unwired: 2 in, 3 out]
            n195 = invoke class="VI" method="Run VI"(reference=w383, error in=w387, "Wait until done"=FALSE ("结束前等待"), "Auto Dispose Ref"=TRUE ("自动销毁引用")) -> (error out=w384:errorcluster)  [unwired: 1 in, 4 out]
          }
          frame Disabled {
            n196 = vi-ref "Auto.vi"() -> (w389:refnum<vi>)
            n197 = call "CallVI.vi"("VI引用"=w389, "状态"=T3."Maximized") -> ()  [unwired: 12 in, 2 out]
          }
        }
        n198 = call <vilib>:"Add State(s) to Queue__jki_lib_state_machine.vi"("State(s) in (\"\")"=w381) -> ("States Out"=w380:string)  [unwired: 14 in]
      }
      frame "UI: Init" {
        n199 = stacked-sequence {
          tunnel: w391 -> [_ _ _ _]
          frame #0 {
            n200 = global write "Global.vi" "程序关闭"(FALSE ("程序关闭")) -> ()
            n201 = control-ref of="电流特性"() -> (w400:refnum<vi>)
            n202 = control-ref of="轴承压装"() -> (w403:refnum<vi>)
            n203 = control-ref of="端铆"() -> (w401:refnum<vi>)
            n204 = control-ref of="侧铆"() -> (w402:refnum<vi>)
            n205 = global write "A180648.vi" "LED-轴承压装"(w403) -> ()
            n206 = global write "A180648.vi" "LED-电流特性"(w400) -> ()
            n207 = global write "A180648.vi" "LED-侧铆"(w402) -> ()
            n208 = global write "A180648.vi" "LED-端铆"(w401) -> ()
            n209 = control-ref of="逆向空载"() -> (w399:refnum<vi>)
            n210 = control-ref of="振动NVH"() -> (w397:refnum<vi>)
            n211 = control-ref of="传感器特性"() -> (w398:refnum<vi>)
            n212 = control-ref of="磨合"() -> (w396:refnum<vi>)
            n213 = global write "A180648.vi" "LED-传感器特性"(w398) -> ()
            n214 = global write "A180648.vi" "LED-逆向空载"(w399) -> ()
            n215 = global write "A180648.vi" "LED-振动NVH"(w397) -> ()
            n216 = global write "A180648.vi" "LED-磨合"(w396) -> ()
          }
          frame #1 {
            w411 = 0
            n217 = shared-variable "我的电脑\\Global.lvlib\\总成追溯码"("   " ("工位追溯码")) -> ()  [unwired: 1 in, 1 out]
            n218 = global write "Global.vi" "生产数量"(w411) -> ()
            n219 = global write "Global.vi" "合格数量"(w411) -> ()
            n220 = global read "Global.vi" "用户信息"() -> (w408:T9)
            n221 = global read "Global.vi" "联机模式"() -> (w405:enum16{"单机", "追溯"})
            n222 = Unbundle By Name(w408) -> ("用户名"=→"userName":string, "用户权限"=→"userStatus":string)
            n223 = case shown="\"追溯\"" w405 {
              tunnel: ["联网" ("connectionMode") "单机" ("connectionMode")] -> w412
              frame "追溯" {
              }
              frame "单机", Default {
              }
            }
            "connectionMode" <- w412
            "产品型号" <- "" ("产品型号")
          }
          frame #2 {
            n224 = control-ref of="提示信息"() -> (w417:refnum<vi>)
            n225 = control-ref of="自动"() -> (w418:refnum<vi>)
            n226 = control-ref of="错误"() -> (w419:refnum<vi>)
            n227 = control-ref of="Result"() -> (w420:refnum<vi>)
            n228 = control-ref of="更换产品"() -> (w416:refnum<vi>)
            n229 = global write "Global.vi" "提示信息"(w417) -> ()
            n230 = global write "Global.vi" "程序自动"(w418) -> ()
            n231 = global write "Global.vi" "报警图标"(w419) -> ()
            n232 = global write "Global.vi" "Result"(w420) -> ()
            n233 = global write "Global.vi" "更换产品"(w416) -> ()
            n234 = control-ref of="状态"() -> (w415:refnum<vi>)
            n235 = global write "Global.vi" "状态"(w415) -> ()
          }
          frame #3 {
            n236 = global read "Global.vi" "Result"() -> (w423:refnum<vi>)
            n237 = property class="Tbl"(reference=w423, "Row Headers[]"=string[] [], "Value"=string[][] []) -> ()  [unwired: 1 in, 2 out]
            n238 = call "Start_Client.vi"() -> ()  [unwired: 12 in]
          }
        }
        n239 = call <vilib>:"Add State(s) to Queue__jki_lib_state_machine.vi"("State(s) in (\"\")"=w395) -> ("States Out"=w394:string)  [unwired: 14 in]
      }
      frame "UI: Config" {
        n240 = vi-ref "Config.vi"() -> (w426:refnum<vi>)
        n241 = call "CallVI.vi"("VI引用"=w426, "状态"=T3."Standard") -> ()  [unwired: 12 in, 2 out]
        n242 = call <vilib>:"Add State(s) to Queue__jki_lib_state_machine.vi"("State(s) in (\"\")"=w431) -> ("States Out"=w430:string)  [unwired: 14 in]
      }
      frame "UI: Cursor Set" {
        # "Argument"
        n243 = case shown="\"Idle\", 默认" w434 {
          tunnel: w436 -> [w441 w443]
          tunnel: [w440 w442] -> w435
          frame "Idle", Default {
            n244 = call <vilib>:"Unset Busy.vi"("error in (no error)"=w441) -> ("error out"=w440:errorcluster)  [unwired: 10 in]
          }
          frame "Busy" {
            n245 = call <vilib>:"Set Busy.vi"("error in (no error)"=w443) -> ("error out"=w442:errorcluster)  [unwired: 9 in, 1 out]
          }
        }
        n246 = call <vilib>:"Add State(s) to Queue__jki_lib_state_machine.vi"("State(s) in (\"\")"=w439) -> ("States Out"=w438:string)  [unwired: 14 in]
      }
      frame "UI: Front Panel State" {
        # "Argument"
        n247 = Unbundle By Name(w448) -> ("Core.Current VI Reference"=w447:refnum<vi>)
        n248 = case shown="\"Close\"" w446 {
          tunnel: w450 -> [w456 w469]
          tunnel: [w458 w470] -> w449
          tunnel: w447 -> [w457 w467]
          frame "Open", Default {
            n249 = property class="VI"(reference=w457, error in=w456) -> (reference out=w454:refnum<vi>, error out=w455:errorcluster, "Front Panel.Open"=w453:bool)
            n250 = case shown="假" w453 {
              tunnel: [w461 w464] -> w458
              tunnel: w455 -> [w460 w464]
              tunnel: w454 -> [w459 _]
              frame False {
                n251 = invoke class="VI" method="FP.Open"(reference=w459, error in=w460, "Activate"=TRUE, "State"=T3."Standard") -> (error out=w461:errorcluster)  [unwired: 1 in, 4 out]
              }
              frame True {
              }
            }
          }
          frame "Close" {
            n252 = property class="VI"(reference=w467, error in=w469) -> (reference out=w466:refnum<vi>, error out=w468:errorcluster, "Front Panel.Open"=w465:bool)
            n253 = case shown="真" w465 {
              tunnel: [w471 w474] -> w470
              tunnel: w468 -> [w471 w473]
              tunnel: w466 -> [_ w472]
              frame False {
              }
              frame True {
                n254 = invoke class="VI" method="FP.Close"(reference=w472, error in=w473) -> (error out=w474:errorcluster)  [unwired: 1 in, 2 out]
              }
            }
          }
        }
        n255 = call <vilib>:"Add State(s) to Queue__jki_lib_state_machine.vi"("State(s) in (\"\")"=w452) -> ("States Out"=w451:string)  [unwired: 14 in]
      }
      frame "---------- Macro ----------" {
        n256 = call <vilib>:"Add State(s) to Queue__jki_lib_state_machine.vi"("State(s) in (\"\")"=w480) -> ("States Out"=w479:string)  [unwired: 14 in]
      }
      frame "Macro: Initialize" {
        n257 = call <vilib>:"Add State(s) to Queue__jki_lib_state_machine.vi"("State(s) in Front (\"\")"="Data: Initialize\nInitialize Core Data\nS7: Initialize\nIdle\nUI: Init\nUI: Front Panel State >> Open\nUI: Initialize\nUI: Config", "State(s) in (\"\")"=w487) -> ("States Out"=w486:string)  [unwired: 13 in]
      }
      frame "Macro: Exit" {
        n258 = Unbundle By Name(w496) -> ("Core.Close Panel on Exit?"=w495:bool)
        n259 = Select(t="UI: Front Panel State >> Close", s=w495, f="") -> (s? t:f=w492:string)
        n260 = call <vilib>:"Add State(s) to Queue__jki_lib_state_machine.vi"("State(s) in (\"\")"=w492, "State(s) at Back (\"\")"="Data: Cleanup\nExit") -> ("States Out"=w490:string)  [unwired: 13 in]
        n261 = call <vilib>:"Add State(s) to Queue__jki_lib_state_machine.vi"("State(s) in Front (\"\")"=w490, "State(s) in (\"\")"=w499) -> ("States Out"=w498:string)  [unwired: 13 in]
      }
    }
  }
  n262 = call-dynamic "Cleanup.vi"("MenuStrip in"=w6) -> ()  [unwired: 10 in, 1 out]
